vi "gyro-V5.vi"() -> ()   [LabVIEW 2017]
uses:
  lorentzian.ctl
  circle corners.ctl
  <vilib>/event_ctls.llb/eventvkey.ctl
  peak -- parameters -- complex fit.ctl
  wavepacket.ctl
  filter method control.ctl
  cursor winow.ctl
  parameters -- scan monitor control.ctl
  pid -- parameters.ctl
  agregator -- action.ctl
  filename-pattern.ctl
  plot refs -- filter related.ctl
  cursor window action.ctl
  cursor action.ctl
  KM_file -- read-write control.ctl
  filename-action.ctl
  publisher action.ctl
  MFLI controller action.ctl
  sweep parameters.ctl
  file -- read-write control.ctl
  <vilib>/Analysis/baseanly.llb/A x B.vi
  <vilib>/Analysis/baseanly.llb/Complex A x B.vi
  line -- complex.vi
  Q -- check range -- i -- integer.vi
  linear interpolation - real.vi
  linear interpolation iiii- complex.vi
  Q - not nan -- real.vi
  filter - complex - four.vi
  peak -- PM find lorenzian - V3.vi
  Q - not nan -- integer.vi
  tale of three indices.vi
  filter -- window span logic.vi
  linear interp iiii- complex - z-omega - divide.vi
  containing bix.vi
  peak -- guess at omega -- dzdomega V2.vi
  command stack.vi
  tale of three indices -- check state.vi
  peak -- z center from mult phase points.vi
  peak -- estimate for lorentzian.vi
  peak -- fake phase around center.vi
  peak -- get weights.vi
  peak -- four corner circle transformation logic.vi
  peak - fit phase around center - V2.vi
  array - generate range.vi
  circle center from three points.vi
  <vilib>/Utility/error.llb/Clear Errors.vi
  <vilib>/Analysis/Matrix/Numeric/Conversions/Array To Matrix.vi
  <vilib>/Analysis/Matrix/Numeric/Conversions/Array To Matrix - RA2.vi
  <vilib>/Analysis/baseanly.llb/Inverse Matrix.vi
  <vilib>/Analysis/baseanly.llb/Real Inverse Matrix.vi
  peak -- fit function -- minus arctan.vi
  <vilib>/gmath/NumericalOptimization/Nonlinear Curve Fit.vi
  <vilib>/gmath/NumericalOptimization/Nonlinear Curve Fit LM.vi
  KM_filter pipe - plot staff - more - V3.vi
  four-corner circle transformation.ctl
panel:
  out "read freq (Hz)":dbl=43834.543279430705 format="%-#11_11f"
  in  "all":enum32{"all", "other"}(tab)
  in  "subtract bgnd !":bool=TRUE
  out "angle (deg)":dbl format="%#11_11f"
  out "Temperature (K)":dbl=49.92548 format="%#11_11f"
  out "Field (T)":dbl=12.0 format="%#11_11f"
  out "Plot: circle sweep window":cluster{"all rows":dbl[], "all rows":dbl[]}[](graph)
  out "Plot: frequency shift vs T":cluster{dbl[], dbl[]}(graph)
  in  "MFLI mode":T1(tab)
  out "fit is fine":bool=TRUE
  in  "gamma factor":dbl=1.6
  in  "Auto-update sweep window!":bool
  in  "scan type":enum16{"linear", "arctan"}(ring)
  in  "N":i64=257
  out "sweep time (sec)":dbl=0.07489956999779679
  in  "control sweep!":bool
  out "circle frequency (Hz)":dbl=1234494.459530083 format="%#11_11f"
  out "circle gamma (Hz)":dbl=51497.57560712996 format="%#11_11f"
  out "circle phase (rad)":dbl=2.6250942279275566 format="%#11_11f"
  out "circle Q":dbl=23.971894695546876 format="%#11_11f"
  in  "history length":i32=5
  in  "delay-circle(msec)":i64
  out "read Voltage (V)":cdb=8.437092120710226e-06+0.006122499694529841i format="%#10_10f"
  in  "read !":bool
  out "read Voltage X (V)":dbl=8.437092120710226e-06 format="%#11_11f"
  out "read Voltage Y (V)":dbl=0.006122499694529841 format="%#11_11f"
  in  "delay-read (msec)":i64=300
  in  "read file":path=path "/Users/arkady/Desktop/local_data/Dec2017--preparing-for-Hybrid/sp030_122217.ASC"
  in  "read from disk":bool
  in  "reqested size":i64=30
  in  "refresh":bool=TRUE
  in  "PID parameters":T2={"P (sec)"=60.0, "I (sec)"=10.0}
  in  "save data":enum32{"save", "save num to dropbox"}(tab)
  out "data name pattern":T3={"prefix"="_empty_lever_", "group"="d"}
  out "freqsweep pattern":T3={"prefix"="lsco2", "group"="f"}
  in  "save data ?":bool
  in  "data file name":string="d001_empty_lever_122317.dat"
  in  "Save folder":path=path "/Users/arkady/Downloads"
  in  "freq sweep file name":string="f027_lsco2_122317.dat"
  in  "save number to dropbox":enum32{"save", "do not save"}(tab)
  in  "read file name":string="r003_silicon_empty_lever_122017.dat"
  in  "Save read folder":path=path "/Users/arkady/Downloads"
  out "left freq (Hz)":dbl=1189281.7830129303
  out "right freq (Hz)":dbl=1228830.8938969919
  in  "horisontal axis":enum16{"Time", "temperature", "field", "angle"}(ring)=enum."temperature"
  in  "vertical axis":T4(ring)
  out "center freq (Hz)":dbl=1209056.338454961
  out "window  (Hz)":dbl=39549.11088406133
  in  "talk to MFLI !":bool=TRUE
  in  "plot frequency shift":enum32{"plot"}(tab)
  in  "Plot frequency shift":bool
  in  "aggregate every # sec":dbl=1.0
  in  "plot length (min)":dbl=100.0
  out "Plot: frequency shift vs T 4":cluster{dbl[], dbl[]}(graph)
  out "Plot: frequency shift vs T 5":cluster{i32[], "Array":dbl[]}(graph)
  out "Plot: frequency shift vs T 2":cluster{dbl[], dbl[]}(graph)={[-1.2847105611270713e-06, -8.96090687489996e-07, -1.1878113186140714e-06, -1.0577364834927965e-06, -1.5485833177118755e-06, -1.2397929198806674e-06, -1.3595641386431873e-06, -1.95544238796184e-06, -1.8034552812236216e-06, -2.179156763955588e-06, -3.122427320687229e-06, -2.8927681404839808e-06, -3.2606669096266067e-06, -3.4335859766558394e-06, -4.275106687632253e-06, -4.265556221219542e-06, -4.306275487364196e-06, -5.474328117771029e-06, -5.250873166830706e-06, -6.158584714145268e-06, -6.308121182987117e-06, -6.715358985348123e-06, -7.0693959466281e-06, -7.254226550276167e-06, -7.471558204043555e-06, -8.180360377818478e-06, -8.644635949920024e-06, -9.450401470204308e-06, -1.0542161519072343e-05, -1.0662496796273006e-05, -1.1774006071250966e-05, -1.2809682001462881e-05, -1.3388752026600543e-05, -1.3901539528835397e-05, -1.577875366340369e-05, -1.6275815692673765e-05, -1.7367311318108792e-05, -1.8322241284696204e-05, -1.939577161026033e-05, -2.115027501101159e-05, -2.206547957836183e-05, -2.280844162782534e-05, -2.4123185115153962e-05, -2.3719380386582883e-05, -2.1949158634554497e-05, -1.7482795415692865e-05, -1.190476009852551e-05, -3.0012581586913445e-06, 6.6591691413936944e-06, 1.4913986718231652e-05, 2.1608211101800334e-05, 2.4441429222012755e-05, 2.5496538170609067e-05, 2.5006558977858244e-05, 2.47084954682896e-05, 2.3205579756867926e-05, 2.2241491423599197e-05, 2.059353741490501e-05, 1.940930308820722e-05, 1.8035523877789703e-05, 1.6795019444131693e-05, 1.6233689318685545e-05, 1.530601912625958e-05, 1.471481346136583e-05, 1.3668746476334144e-05, 1.278914735524648e-05, 1.1961636965375277e-05, 1.148511101983816e-05, 1.038015177533868e-05, 1.055813470630652e-05, 8.946114686992878e-06, 9.252763324432675e-06, 9.261580911233215e-06, 8.32864546005932e-06, 7.550850612980853e-06, 7.659009848135973e-06, 6.564878336519785e-06, 6.828313841636074e-06, 6.028961228097367e-06, 6.074863784114649e-06, 5.087873216594783e-06, 5.533364081213274e-06, 5.085350335296872e-06, 4.637182878582281e-06, 4.339275810721466e-06, 3.7404983334720106e-06, 3.8016720277973716e-06, 2.9030355925414103e-06, 3.3221723271601737e-06, 2.724834743267001e-06, 3.0361409970562057e-06, 2.469938271454002e-06, 2.1916218680781524e-06, 1.473344438791089e-06, 1.5465747082434236e-06, 1.5291782659004455e-06, 1.3674315612440997e-06, 9.633298642757269e-07, 8.898825337811226e-07], [-5.351696133733621e-06, -3.690354306686691e-06, -3.6817845026587138e-06, -3.6304954766072717e-06, -3.2238464103788782e-06, -3.732378935963822e-06, -3.493875482979771e-06, -3.3228636578776652e-06, -3.5305288089255853e-06, -3.7648610315931326e-06, -3.97228399037134e-06, -3.69199555481082e-06, -3.702050829314118e-06, -3.6362897452965515e-06, -4.059309516809881e-06, -3.708125867376757e-06, -3.8934710007503085e-06, -3.920425505771773e-06, -3.8396731962881915e-06, -4.145539651931423e-06, -4.426868555366925e-06, -5.042368648209767e-06, -4.738746005563639e-06, -4.890549160081816e-06, -5.391544637503511e-06, -5.223768648790353e-06, -5.325388776256424e-06, -5.912529897926599e-06, -6.493781160800396e-06, -6.198776272723992e-06, -7.250361850269486e-06, -7.26192304305288e-06, -7.774332746184141e-06, -8.356818571969059e-06, -9.494659847987037e-06, -9.933186332652295e-06, -1.0866378585117719e-05, -1.2559721845876861e-05, -1.4157112461896858e-05, -1.656537642835046e-05, -1.936170396817286e-05, -2.2793543082063973e-05, -2.6692434310764325e-05, -3.194302075894453e-05, -3.767957435737811e-05, -4.424063928058543e-05, -4.980677556288027e-05, -5.2904900834404434e-05, -5.2259193151987076e-05, -4.837844245967899e-05, -4.2136497452806694e-05, -3.570466251887759e-05, -3.0332314166196737e-05, -2.6071508393447144e-05, -2.1180215381563472e-05, -1.8286542839044908e-05, -1.61637622680976e-05, -1.3625750559341328e-05, -1.2108594610162641e-05, -1.0689795144437375e-05, -9.62045281676502e-06, -8.570007528029048e-06, -8.105558082533694e-06, -7.428892434368157e-06, -7.218695867625404e-06, -6.953805415589833e-06, -5.913334865014344e-06, -6.088309429175753e-06, -5.145987374849902e-06, -5.488187006895521e-06, -5.163517414643828e-06, -5.079842929772351e-06, -5.245282954840261e-06, -4.660283528196666e-06, -4.4589258860321075e-06, -4.13807438954911e-06, -4.565262237593832e-06, -4.053552425555827e-06, -3.4974249873645082e-06, -3.913051273651945e-06, -3.89264048603008e-06, -3.6773922014571442e-06, -3.2426624479706957e-06, -3.419821634783878e-06, -3.3651012599037013e-06, -3.573387544637086e-06, -4.131232704147514e-06, -3.2305802189117116e-06, -3.021417984572191e-06, -3.2398605602097806e-06, -3.508439835095558e-06, -3.546989372643574e-06, -3.729083758383661e-06, -3.2473817592994867e-06, -3.29870731020323e-06, -3.3620259083252726e-06, -3.419602935105049e-06, -4.225308611898116e-06, -3.737346070152369e-06]}
  out "Plot: frequency shift vs T 3":cluster{i32[], dbl[]}(graph)={[0, 1, 2, 3, 4, 5, 6, 7, 8, 9, 10, 11, 12, 13, 14, 15, 16, 17, 18, 19, 20, 21, 22, 23, 24, 25, 26, 27, 28, 29, 30, 31, 32, 33, 34, 35, 36, 37, 38, 39, 40, 41, 42, 43, 44, 45, 46, 47, 48, 49, 50, 51, 52, 53, 54, 55, 56, 57, 58, 59, 60, 61, 62, 63, 64, 65, 66, 67, 68, 69, 70, 71, 72, 73, 74, 75, 76, 77, 78, 79, 80, 81, 82, 83, 84, 85, 86, 87, 88, 89, 90, 91, 92, 93, 94, 95, 96, 97, 98], [-0.23559860043831193, -0.23820939062512414, -0.3120762913359678, -0.2835001183703665, -0.44780658796424877, -0.32070526654251785, -0.37109881260414546, -0.5319066481282504, -0.4722639722623221, -0.524696373474268, -0.6661788735811576, -0.6646137200418041, -0.7220903993361305, -0.7567345405074919, -0.8112846755002696, -0.8551933851256885, -0.8356992634466227, -0.9493152294582043, -0.9394070576242828, -0.9783311582294316, -0.9588814811243913, -0.9267379794474269, -0.9802698763137818, -0.9776201855738149, -0.9457143265769079, -1.0024951473096775, -1.0186705422504727, -1.0117383851591542, -1.0187082032726575, -1.0441935724590885, -1.0188444902666154, -1.0550639642963695, -1.0447176937736993, -1.0295365240674577, -1.0291006014399389, -1.0228351916589804, -1.0117082035896368, -0.9698748205564658, -0.9402791409053437, -0.9063694667492768, -0.8505714661765986, -0.7857248716608289, -0.7348809545553663, -0.6387178563870073, -0.5274684440579174, -0.37634000181515215, -0.2346170964234171, -0.05666856473380277, 0.12674275046362427, 0.29903345155814187, 0.4738466551438263, 0.6002776366427447, 0.6989959497442624, 0.7645517375308588, 0.8621349432337582, 0.9034008935958421, 0.9423491262817814, 0.9862736125756424, 1.0130206638602015, 1.035756014091886, 1.050605066301123, 1.0850669404773998, 1.083776083480046, 1.1032698129216518, 1.0849090392836143, 1.0727819505921015, 1.1116722316992618, 1.0833561407376393, 1.1105523962821076, 1.0914293641785555, 1.0473253514157124, 1.0687148941515687, 1.0554881441119783, 1.060651558581904, 1.0373768137660564, 1.0754397797680961, 0.9631595802552361, 1.0350672662925295, 1.0451346582720782, 0.9985529870514799, 0.9177123734459048, 0.984236082337904, 1.0031536192825101, 0.9353574049208152, 0.9111749823496003, 0.8082426158031351, 0.7438785320162125, 0.7320472832267922, 0.8327734332640132, 0.6992660900455262, 0.7133566540037093, 0.6082706202737593, 0.5313341296869087, 0.42592845813496805, 0.438412524592966, 0.42687019592046394, 0.38040311101033075, 0.22415893312212232, 0.2337528615998219]}
  in  "aggregator action":T5
  in  "Tab : everything":T6(tab)
  in  "Tab :  Fit controls":enum32{"complex plane", "complex plane 2"}(tab)
  in  "some":dbl=3172.0
  in  "Plot: fragment - filter":cluster{dbl[], dbl[]}[](graph)=[{array[18251 elements], array[18251 elements]}, {array[18251 elements], array[18251 elements]}, {array[18251 elements], array[18251 elements]}, {array[18251 elements], array[18251 elements]}]
  in  "scale gauge: Plot: complex plane - filter":dbl(slide)=0.00015000000000000001 min=0.0 max=0.3 step=1e-05 scale=0.0001..0.3 scale format="%#_5g"
  in  "Plot: complex plane - filter":cluster{dbl[], dbl[]}[](graph)=[{array[18251 elements], array[18251 elements]}, {array[18251 elements], array[18251 elements]}, {[1.0902546658046695e-05, 1.0889761640892542e-05, 1.0851457046051869e-05, 1.078778404426081e-05, 1.0698993923768004e-05, 1.058543709861469e-05, 1.044756172571057e-05, 1.0285911936163232e-05, 1.0101125687841252e-05, 9.89393224764595e-06, 9.6651493134281e-06, 9.41567978690808e-06, 9.146508210335277e-06, 8.858696880949628e-06, 8.55338165857973e-06, 8.231767482923022e-06, 7.895123618199276e-06, 7.5447786439446085e-06, 7.182115211715007e-06, 6.808564588392319e-06, 6.425601007627753e-06, 6.03473585171517e-06, 5.637511686855652e-06, 5.235496175353443e-06, 4.830275888769022e-06, 4.423450046446e-06, 4.016624204122979e-06, 3.6114039175385575e-06, 3.209388406036347e-06, 2.81216424117683e-06, 2.4212990852642467e-06, 2.038335504499682e-06, 1.6647848811769937e-06, 1.3021214489473908e-06, 9.517764746927217e-07, 6.151326099689789e-07, 2.935184343122684e-07, -1.1796788057628133e-08, -2.996081174432771e-07, -5.687796940160799e-07, -8.182492205360993e-07, -1.047032154753949e-06, -1.2542255949492504e-06, -1.439011843271231e-06, -1.6006616328185704e-06, -1.73853700572269e-06, -1.8520938308760026e-06, -1.9408839513688086e-06, -2.0045569531598684e-06, -2.0428615480005406e-06, -2.055646565154694e-06, -2.0428615480005406e-06, -2.0045569531598684e-06, -1.9408839513688077e-06, -1.8520938308760026e-06, -1.7385370057226892e-06, -1.6006616328185688e-06, -1.43901184327123e-06, -1.2542255949492496e-06, -1.0470321547539481e-06, -8.182492205360985e-07, -5.687796940160773e-07, -2.9960811744327624e-07, -1.1796788057627286e-08, 2.935184343122701e-07, 6.151326099689776e-07, 9.517764746927255e-07, 1.3021214489473916e-06, 1.664784881176997e-06, 2.038335504499683e-06, 2.4212990852642467e-06, 2.812164241176833e-06, 3.2093884060363485e-06, 3.6114039175385617e-06, 4.01662420412298e-06, 4.423450046446e-06, 4.8302758887690245e-06, 5.235496175353443e-06, 5.637511686855656e-06, 6.034735851715172e-06, 6.425601007627752e-06, 6.8085645883923205e-06, 7.182115211715006e-06, 7.544778643944612e-06, 7.895123618199278e-06, 8.231767482923025e-06, 8.553381658579734e-06, 8.858696880949628e-06, 9.146508210335279e-06, 9.41567978690808e-06, 9.665149313428104e-06, 9.893932247645952e-06, 1.0101125687841252e-05, 1.0285911936163232e-05, 1.0447561725710571e-05, 1.0585437098614693e-05, 1.0698993923768004e-05, 1.078778404426081e-05, 1.0851457046051869e-05, 1.0889761640892542e-05], [3.0357756803340517e-06, 3.442601522657073e-06, 3.847821809241494e-06, 4.249837320743704e-06, 4.647061485603221e-06, 5.037926641515804e-06, 5.42089022228037e-06, 5.7944408456030584e-06, 6.1571042778326605e-06, 6.507449252087329e-06, 6.844093116811073e-06, 7.165707292467784e-06, 7.47102251483768e-06, 7.758833844223328e-06, 8.028005420796131e-06, 8.277474947316151e-06, 8.506257881534001e-06, 8.713451321729303e-06, 8.898237570051283e-06, 9.059887359598623e-06, 9.19776273250274e-06, 9.311319557656056e-06, 9.400109678148862e-06, 9.46378267993992e-06, 9.502087274780593e-06, 9.514872291934746e-06, 9.502087274780593e-06, 9.46378267993992e-06, 9.40010967814886e-06, 9.311319557656056e-06, 9.19776273250274e-06, 9.059887359598621e-06, 8.898237570051283e-06, 8.713451321729302e-06, 8.506257881534001e-06, 8.277474947316151e-06, 8.028005420796131e-06, 7.758833844223327e-06, 7.4710225148376794e-06, 7.165707292467782e-06, 6.844093116811075e-06, 6.507449252087329e-06, 6.15710427783266e-06, 5.794440845603057e-06, 5.420890222280368e-06, 5.0379266415158025e-06, 4.647061485603221e-06, 4.249837320743704e-06, 3.847821809241493e-06, 3.4426015226570715e-06, 3.0357756803340496e-06, 2.62894983801103e-06, 2.2237295514266096e-06, 1.8217140399243985e-06, 1.4244898750648805e-06, 1.033624719152297e-06, 6.506611383877313e-07, 2.7711051506504534e-07, -8.55529171645576e-08, -4.3589789141922626e-07, -7.72541756142972e-07, -1.0941559317996812e-06, -1.399471154169577e-06, -1.687282483555225e-06, -1.9564540601280286e-06, -2.205923586648048e-06, -2.4347065208658994e-06, -2.6418999610611992e-06, -2.8266862093831814e-06, -2.9883359989305192e-06, -3.126211371834638e-06, -3.2397681969879523e-06, -3.3285583174807574e-06, -3.3922313192718172e-06, -3.4305359141124894e-06, -3.443320931266643e-06, -3.4305359141124894e-06, -3.3922313192718172e-06, -3.3285583174807565e-06, -3.2397681969879514e-06, -3.126211371834639e-06, -2.9883359989305175e-06, -2.8266862093831797e-06, -2.6418999610611975e-06, -2.434706520865897e-06, -2.2059235866480456e-06, -1.956454060128026e-06, -1.687282483555225e-06, -1.3994711541695744e-06, -1.0941559317996795e-06, -7.72541756142967e-07, -4.358978914192233e-07, -8.555291716455718e-08, 2.771105150650479e-07, 6.506611383877338e-07, 1.033624719152303e-06, 1.4244898750648839e-06, 1.821714039924399e-06, 2.2237295514266125e-06, 2.628949838011031e-06]}, {[-1.0628665430958349e-06, 6.164050781399584e-07, 1.2136346376816573e-06], [-2.749099041575702e-07, -4.987758850147442e-07, 3.798056853807086e-07]}, {[-2.689773598781885e-07, -2.658273840778637e-07, -2.626774082775389e-07, -2.595274324772141e-07, -2.5637745667688934e-07, -2.5322748087656455e-07, -2.5007750507623977e-07, -2.46927529275915e-07, -2.437775534755902e-07, -2.406275776752654e-07, -2.3747760187494066e-07, -2.3432762607461587e-07, -2.311776502742911e-07, -2.280276744739663e-07, -2.2487769867364152e-07, -2.2172772287331676e-07, -2.1857774707299197e-07, -2.154277712726672e-07, -2.122777954723424e-07, -2.0912781967201762e-07], [-2.2381592717709463e-07, -2.1935795690029337e-07, -2.1489998662349214e-07, -2.1044201634669088e-07, -2.0598404606988962e-07, -2.015260757930884e-07, -1.9706810551628713e-07, -1.926101352394859e-07, -1.8815216496268464e-07, -1.8369419468588339e-07, -1.7923622440908216e-07, -1.747782541322809e-07, -1.7032028385547964e-07, -1.658623135786784e-07, -1.6140434330187715e-07, -1.569463730250759e-07, -1.5248840274827466e-07, -1.480304324714734e-07, -1.4357246219467214e-07, -1.3911449191787091e-07]}, {[6.164050781399584e-07, 7.064288860098442e-07, 7.9645269387973e-07, 8.86476501749616e-07, 9.765003096195017e-07, 1.0665241174893877e-06, 1.1565479253592736e-06, 1.2465717332291596e-06, 1.3365955410990453e-06, 1.426619348968931e-06, 1.516643156838817e-06, 1.606666964708703e-06, 1.696690772578589e-06, 1.7867145804484747e-06, 1.8767383883183606e-06, 1.9667621961882463e-06, 2.0567860040581323e-06, 2.1468098119280182e-06, 2.2368336197979038e-06, 2.32685742766779e-06], [-4.987758850147442e-07, -4.987758850147442e-07, -4.987758850147442e-07, -4.987758850147442e-07, -4.987758850147442e-07, -4.987758850147442e-07, -4.987758850147442e-07, -4.987758850147442e-07, -4.987758850147442e-07, -4.987758850147442e-07, -4.987758850147442e-07, -4.987758850147442e-07, -4.987758850147442e-07, -4.987758850147442e-07, -4.987758850147442e-07, -4.987758850147442e-07, -4.987758850147442e-07, -4.987758850147442e-07, -4.987758850147442e-07, -4.987758850147442e-07]}]
  out "Plot: dz/domega":cluster{"omega out":dbl[], dbl[]}(graph)
  out "Plot: win omega":T7(graph)
  out "Plot: phase":cluster{"omega out":dbl[], dbl[]}(graph)
  out "Plot: phase around center":cluster{dbl[], dbl[]}[](graph)
  out "Plot: fragment":cluster{dbl[], dbl[]}[](graph)
  out "Plot: complex plane":cluster{dbl[], dbl[]}[](graph)=[{array[18251 elements], array[18251 elements]}, {[4.093261515777318e-06, 4.09109240444531e-06, 4.084619278630759e-06, 4.073944223394617e-06, 4.059235590734925e-06, 4.040725344575241e-06, 4.018705402554987e-06, 3.993523032313897e-06, 3.965575374873894e-06, 3.9353031814879255e-06, 3.903183862729422e-06, 3.869723959442356e-06, 3.835451154289541e-06, 3.8009059498818182e-06, 3.7666331447290027e-06, 3.7331732414419364e-06, 3.701053922683433e-06, 3.670781729297465e-06, 3.6428340718574613e-06, 3.6176517016163716e-06, 3.5956317595961173e-06, 3.5771215134364333e-06, 3.5624128807767425e-06, 3.5517378255406e-06, 3.5452646997260484e-06, 3.543095588394041e-06, 3.5452646997260484e-06, 3.5517378255406e-06, 3.5624128807767425e-06, 3.5771215134364333e-06, 3.5956317595961173e-06, 3.6176517016163716e-06, 3.6428340718574613e-06, 3.670781729297465e-06, 3.701053922683433e-06, 3.7331732414419364e-06, 3.766633144729003e-06, 3.8009059498818182e-06, 3.835451154289541e-06, 3.869723959442356e-06, 3.903183862729422e-06, 3.9353031814879255e-06, 3.965575374873894e-06, 3.993523032313897e-06, 4.018705402554987e-06, 4.040725344575242e-06, 4.059235590734925e-06, 4.073944223394617e-06, 4.084619278630759e-06, 4.09109240444531e-06], [3.4730573631850562e-06, 3.507534400522981e-06, 3.5414677143865035e-06, 3.574322156145216e-06, 3.605579591626292e-06, 3.634747072399907e-06, 3.661364609870454e-06, 3.6850124295714753e-06, 3.7053175912597633e-06, 3.7219598704057783e-06, 3.734676808325772e-06, 3.7432678513120154e-06, 3.747597513484575e-06, 3.747597513484575e-06, 3.7432678513120154e-06, 3.734676808325772e-06, 3.7219598704057783e-06, 3.7053175912597633e-06, 3.6850124295714753e-06, 3.661364609870454e-06, 3.634747072399907e-06, 3.6055795916262915e-06, 3.574322156145216e-06, 3.5414677143865035e-06, 3.507534400522981e-06, 3.4730573631850562e-06, 3.4385803258471313e-06, 3.404647011983609e-06, 3.371792570224896e-06, 3.3405351347438205e-06, 3.311367653970205e-06, 3.2847501164996586e-06, 3.261102296798637e-06, 3.240797135110349e-06, 3.224154855964334e-06, 3.2114379180443405e-06, 3.202846875058097e-06, 3.1985172128855375e-06, 3.1985172128855375e-06, 3.202846875058097e-06, 3.2114379180443405e-06, 3.224154855964334e-06, 3.240797135110349e-06, 3.2611022967986376e-06, 3.284750116499659e-06, 3.3113676539702056e-06, 3.3405351347438205e-06, 3.3717925702248966e-06, 3.404647011983609e-06, 3.4385803258471313e-06]}, {[3.6823320311784962e-06, 3.6959166832692147e-06, 3.7095013353599328e-06, 3.7230859874506512e-06, 3.7366706395413693e-06, 3.7502552916320878e-06, 3.7638399437228063e-06, 3.7774245958135243e-06, 3.791009247904243e-06, 3.804593899994961e-06, 3.818178552085679e-06, 3.831763204176397e-06, 3.845347856267116e-06, 3.858932508357834e-06, 3.872517160448552e-06, 3.886101812539271e-06, 3.899686464629989e-06, 3.9132711167207074e-06, 3.9268557688114255e-06, 3.940440420902144e-06], [3.233857949158204e-06, 3.257777890560889e-06, 3.2816978319635747e-06, 3.3056177733662597e-06, 3.329537714768945e-06, 3.35345765617163e-06, 3.3773775975743154e-06, 3.4012975389770005e-06, 3.4252174803796856e-06, 3.449137421782371e-06, 3.4730573631850562e-06, 3.4969773045877413e-06, 3.520897245990427e-06, 3.544817187393112e-06, 3.568737128795797e-06, 3.5926570701984825e-06, 3.6165770116011676e-06, 3.6404969530038527e-06, 3.664416894406538e-06, 3.6883368358092233e-06]}, {[3.5789791380588267e-06, 3.602899079461512e-06, 3.6268190208641973e-06, 3.6507389622668824e-06, 3.674658903669568e-06, 3.698578845072253e-06, 3.722498786474938e-06, 3.7464187278776236e-06, 3.7703386692803087e-06, 3.7942586106829942e-06, 3.818178552085679e-06, 3.842098493488365e-06, 3.8660184348910495e-06, 3.889938376293735e-06, 3.9138583176964205e-06, 3.937778259099106e-06, 3.961698200501791e-06, 3.985618141904476e-06, 4.009538083307162e-06, 4.0334580247098464e-06], [3.608903884092239e-06, 3.595319232001521e-06, 3.5817345799108024e-06, 3.568149927820084e-06, 3.554565275729366e-06, 3.5409806236386478e-06, 3.5273959715479293e-06, 3.513811319457211e-06, 3.5002266673664928e-06, 3.4866420152757747e-06, 3.4730573631850562e-06, 3.4594727110943377e-06, 3.4458880590036197e-06, 3.4323034069129016e-06, 3.418718754822183e-06, 3.4051341027314647e-06, 3.3915494506407466e-06, 3.3779647985500286e-06, 3.36438014645931e-06, 3.3507954943685916e-06]}, {[0.11020964852293831, 0.1081676673664668, 0.10605808731817996, 0.10388222679693825, 0.10164144564474008, 0.09933714427686499, 0.09697076280665969, 0.09454378014551397, 0.0920577130785894, 0.08951411531687781, 0.08691457652618259, 0.08426072133362926, 0.0815542083123265, 0.07879672894481177, 0.07599000656593, 0.07313579528580517, 0.0702358788935788, 0.06729206974259966, 0.06430620761776203, 0.06128015858569991], [0.0803136449141255, 0.08304340836327952, 0.08572127459436578, 0.0883455700281582, 0.09091465456543511, 0.09342692261198808, 0.09588080408206583, 0.09827476537962686, 0.10060731035678701, 0.10287698124886316, 0.10508235958542876, 0.10722206707681159, 0.10929476647548003, 0.1112991624117792, 0.11323400220349483, 0.1150980766387388, 0.1168902207316674, 0.1186093144505593, 0.12025428341779912, 0.1218240995813284]}, {[0.12233229108551504, 0.12006569200183163, 0.11772405814823327, 0.11530885296965496, 0.11282158589071498, 0.11026381137237364, 0.10763712794044575, 0.104943177186574, 0.10218364274228772, 0.09936024922678786, 0.09647476116911617, 0.09352898190538197, 0.09052475245173591, 0.08746395035379456, 0.0843484885132358, 0.08118031399229725, 0.07796140679692595, 0.07469377863933911, 0.07137947168076934, 0.06802055725518039], [0.08914775705400713, 0.09217779448256808, 0.09515022599907384, 0.09806319393058342, 0.1009148777669608, 0.10370349529863458, 0.10642730373042088, 0.10908460077071364, 0.11167372569536141, 0.11419306038556593, 0.11664103033915374, 0.11901610565458869, 0.12131680198711066, 0.12354168147640275, 0.12568935364520709, 0.1277584762683279, 0.12974775621147863, 0.13165595023944865, 0.13348186579308485, 0.13522436173460234]}, {array[18251 elements], array[18251 elements]}]
  in  "scale gauge: Plot: complex plane":dbl(slide)=0.00025 min=0.0 max=0.3 step=1e-05 scale=0.0001..1.0 scale format="%#_2g"
  out "window width (kHz)":dbl=76.27809365793496
  out "window center (kHz)":dbl=3399.029286744401
  out "# of points in window":dbl=953.475933538175
  in  "use fast fit?":bool
  out "pm lorentzian":T8={"Amplitude"=0.014166105720943529, "omega(0)"=1234494.459530083, "Gamma"=51497.57560712996, "phase"=2.6250942279275566, "Q"=23.971894695546876, "Norm  Ampl"=nan, "z (inf)"=3.6823320311784962e-06+3.233857949158204e-06i, "4corners"={"z (-pi/2)"=3.5789791380588267e-06+3.608903884092239e-06i, "z(inf)"=3.6823320311784962e-06+3.233857949158204e-06i, "z (pi/2)"=4.057377966112532e-06+3.3372108422778735e-06i, "z center"=3.818178552085679e-06+3.4730573631850562e-06i, "z(0)"=3.9540250729928624e-06+3.7122567772119084e-06i, "radius"=2.750829636916383e-07}} {"z (inf)" format="%#9_9f"; "Q" format="%#9_9f"; "phase" format="%#9_9f"; "Gamma" format="%#9_9f"; "omega(0)" format="%#9_9f"}
  in  "plot staff":enum16{"plot", "do not plot", "a"}(ring)
  in  "fit?":bool=TRUE
  out "Freq out":dbl[](array[numeric])
  out "Voltage out":cdb[](array[numeric])
  in  "cursor bracket: fit boundaries":T10={"left"=1016786.9846609245, "right "=1413121.3581259316, "center"=1214954.171393428, "window"=396334.373465007, "cursors"=[3, 4, 5], "relative"=0, "absolute"=0, "fixed vertical offset"=0.0, "vertical offset"=0.0, "skew"=0.0, "default window frac"=0.1, "kind"=enum."symmetric", "skew.left"=0.5, "skew.right"=0.5, "Plot ref"=refnum, "wing order"=enum."forw"}
  in  "scan monitor control":T11={"gamma acc. frac. - min "=0.3, "gamma acc frac.. - max"=3.0, "peak acc. fraction (af)"=5.0, "min peak acc. window (kHz)"=0.5, "use"=enum."fraction", "abs gamma min(kHz)"=0.005, "abs gamma max(kHz)"=5.0, "# points"=5, "gamma-factor (fa)"=3.0, "interpolate"=enum."line", "init"=TRUE, "Unique strike parameters"=TRUE, "max peak acc. window (kHz)"=10.0, "spacing factor"=1.5, "iterate #"=1, "overwrite ctl?"=FALSE, "write _m files?"=FALSE, "max slope (kHz/sweep)"=0.5, "funnel state"=enum."funnel open"}
  in  "Update system parameters":bool
  in  "parameters: complex fit":T12={"main VI path"=path "", "scale factor"=3.0, "# of grid points"=200, "parameters: wavepacket"={"R"=0.5, "wave number"=22.0, "delta k"=7.0, "radii vector"=[], "radial section"=[], "wave vector"=22.0, "wavepacket is"=TRUE}, "span"=0.27789, "interference ?"=enum."cp z center", "filter method"=enum."three"} {"span" min=0.0 max=0.5 step=1e-05 scale=0.0001..0.5 scale format="%#_5f"; "parameters: wavepacket"."delta k" format="%#_3f"; "parameters: wavepacket"."wave number" format="%#_3f"; "parameters: wavepacket"."R" format="%#_3f"}
  in  "cursor bracket: circle window":T10={"left"=1189281.7830129303, "right "=1228830.8938969919, "center"=1209056.338454961, "window"=39549.11088406133, "cursors"=[0, 1, 2], "relative"=1, "absolute"=1, "fixed vertical offset"=0.0, "vertical offset"=0.0, "skew"=0.0, "default window frac"=0.1, "kind"=enum."symmetric", "skew.left"=0.5, "skew.right"=0.5, "Plot ref"=refnum, "wing order"=enum."forw"}
  in  "Tab : parameters":enum32{"Page 1"}(tab)
  out "VKey":T15
  out "Char":i16=45
  # "three strikes"
  # "search window"
  # "linear extrapolation"
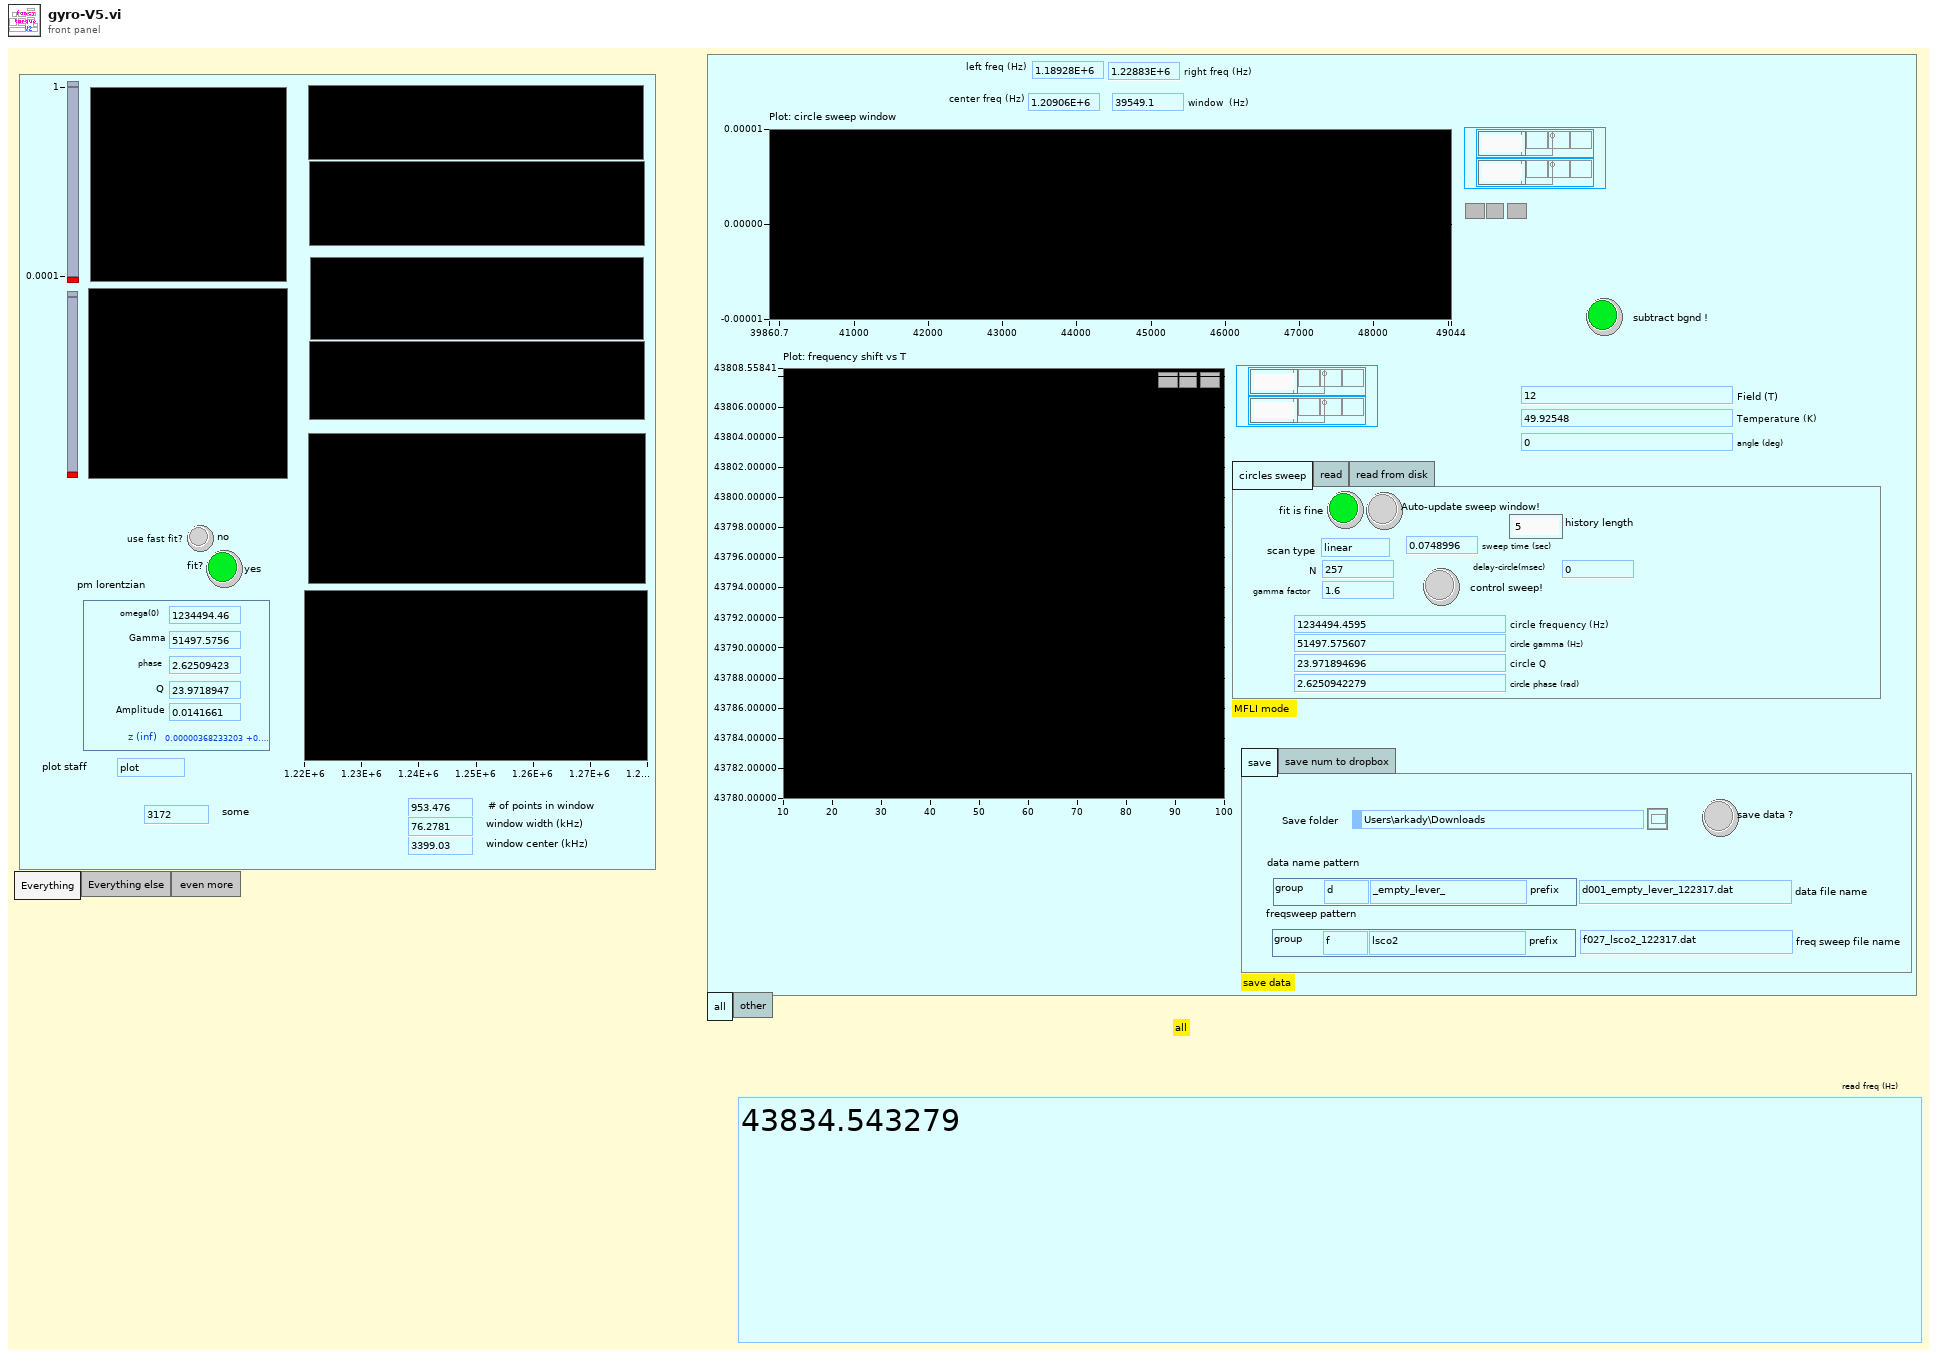
[diagram p1: front panel]
types:
  T1 = enum32{"circles sweep", "read", "read from disk", "circle PLL"}
  T2 = typedef "pid -- parameters.ctl" = cluster{"P (sec)":dbl, "I (sec)":dbl}
  T3 = typedef "filename-pattern.ctl" = cluster{"prefix":string, "group":string}
  T4 = enum16{"frequency", "gamma", "phase", "background"}
  T5 = typedef "agregator -- action.ctl" = enum16{"append", "interpolate", "empty!", "force", "init", "scale", "read last"}
  T6 = enum32{"Everything", "Everything else", "even more "}
  T7 = cluster{"omega out":dbl[], "win omega out":dbl[]}
  T8 = typedef "lorentzian.ctl" = cluster{"Amplitude":dbl, "omega(0)":dbl, "Gamma":dbl, "phase":dbl, "Q":dbl, "Norm  Ampl":dbl, "z (inf)":cdb, "4corners":T9}
  T9 = typedef "circle corners.ctl" = cluster{"z (-pi/2)":cdb, "z(inf)":cdb, "z (pi/2)":cdb, "z center":cdb, "z(0)":cdb, "radius":dbl}
  T10 = typedef "cursor winow.ctl" = cluster{"left":dbl, "right ":dbl, "center":dbl, "window":dbl, "cursors":i32[], "relative":i32, "absolute":i32, "fixed vertical offset":dbl, "vertical offset":dbl, "skew":dbl, "default window frac":dbl, "kind":enum16{"symmetric", "skewed", "fancy"}, "skew.left":dbl, "skew.right":dbl, "Plot ref":refnum<vi>, "wing order":enum16{"forw", "back"}}
  T11 = typedef "parameters -- scan monitor control.ctl" = cluster{"gamma acc. frac. - min ":dbl, "gamma acc frac.. - max":dbl, "peak acc. fraction (af)":dbl, "min peak acc. window (kHz)":dbl, "use":enum16{"window", "fraction"}, "abs gamma min(kHz)":dbl, "abs gamma max(kHz)":dbl, "# points":i32, "gamma-factor (fa)":dbl, "interpolate":enum16{"line", "last"}, "init":bool, "Unique strike parameters":bool, "max peak acc. window (kHz)":dbl, "spacing factor":dbl, "iterate #":i32, "overwrite ctl?":bool, "write _m files?":bool, "max slope (kHz/sweep)":dbl, "funnel state":enum16{"funnel open", "funnel closed"}}
  T12 = typedef "peak -- parameters -- complex fit.ctl" = cluster{"main VI path":path, "scale factor":dbl, "# of grid points":i32, "parameters: wavepacket":T13, "span":dbl, "interference ?":enum16{"cp z center", "pm zcenter", "fancy"}, "filter method":T14}
  T13 = typedef "wavepacket.ctl" = cluster{"R":dbl, "wave number":dbl, "delta k":dbl, "radii vector":dbl[], "radial section":cdb[], "wave vector":dbl, "wavepacket is":bool}
  T14 = typedef "filter method control.ctl" = enum16{"four", "five", "one", "two", "three", "zero", "minus one", "minus two"}
  T15 = typedef "eventvkey.ctl" = enum16{"ASCII", "Enter", "Return", "Shift", "Ctrl", "Alt", "Cmd", "Opt", "Caps", "NumLock", "Clear", "Break", "Up", "Down", "Left", "Right", "Insert", "Delete", "Home", "End", "PageUp", "PageDown", "Escape", "Help", "Pause", "ScrollLock", "F1", "F2", "F3", "F4", "F5", "F6", "F7", "F8", "F9", "F10", "F11", "F12", "F13", "F14", "F15", "F16", "F17", "F18", "F19", "F20", "F21", "F22", "F23", "F24", "Play", "VolumeUp", "VolumeDown", "Mute", "Two Byte Char"}
  T16 = typedef "cursor window action.ctl" = enum16{"balance", "h. offset change", "cursor moves", "change center", "change window", "init", "check", "reset", "set y to middle", "idle", "-write all Y", "-write left.X", "-write center.X", "-write right.X", "-write all X", "-change center", "-change window", "-change skew", "-read cursor 2", "-read cursor 1", "-read cursor 0", "-read all cursors", "-reset", "-read plot scale", "-set y to middle", "-Q: center.Y is visible", "-Q: window is visible", "-parse center.Y", "-right left from center", "-left move", "-right move", "-set center.Y", "-empty", "-set cursors to default", "-check", "-write center.Y", "-copy cursor 1", "-copy cursor 0", "-copy cursor 2", "move right", "move left", "shrink", "broaden", "skew up", "skew down", "-write plot scale", "zoom X", "change cen&win", "zoom to all data", "color--red", "color--green", "color--yellow", "read", "zoom out", "zoom in", "slide right", "slide left"}
  T17 = typedef "plot refs -- filter related.ctl" = cluster{"Plot: complex plane - filter":refnum<vi>, "Plot: dz/domega":refnum<vi>, "Plot: fragment filter":refnum<vi>, "Plot: win omega":refnum<vi>, "Plot: phase":refnum<vi>, "Plot: phase around center":refnum<vi>, "Plot: complex plane":refnum<vi>, "Plot: fragment":refnum<vi>}
  T18 = typedef "MFLI controller action.ctl" = enum16{"Initialize", "Scan frequency", "open", "close", "read", "circle PLL"}
  T19 = typedef "file -- read-write control.ctl" = enum16{"read", "write all", "append one line"}
  T20 = typedef "sweep parameters.ctl" = cluster{"scan type":enum16{"linear", "arctan"}, "N":i64, "cursor window":T10}
  T21 = typedef "cursor action.ctl" = enum16{"range", "read", "write", "check", "zoom out", "smart zoom out"}
  T22 = typedef "KM_file -- read-write control.ctl" = enum16{"read", "write all", "append one line"}
  T23 = typedef "filename-action.ctl" = enum16{"rewrite", "parse"}
  T24 = typedef "publisher action.ctl" = enum16{"set", "get"}
  T25 = typedef "four-corner circle transformation.ctl" = enum16{"z(c) z(inf)", "z(c) z(zero)", "fix phase", "calculate lorentzian", "z(0) z(+-pi/2)", "shift to zcenter", "to  canonical", "get canonical phase", "get4corners"}
  T26 = typedef "interpolation state - real.ctl" = cluster{"requested size":i32, "Array":dbl[], "actual number of elements":i32}
  T27 = typedef "interpolation state - complex.ctl" = cluster{"requested size":i32, "Array":cdb[], "actual number of elements":i32}
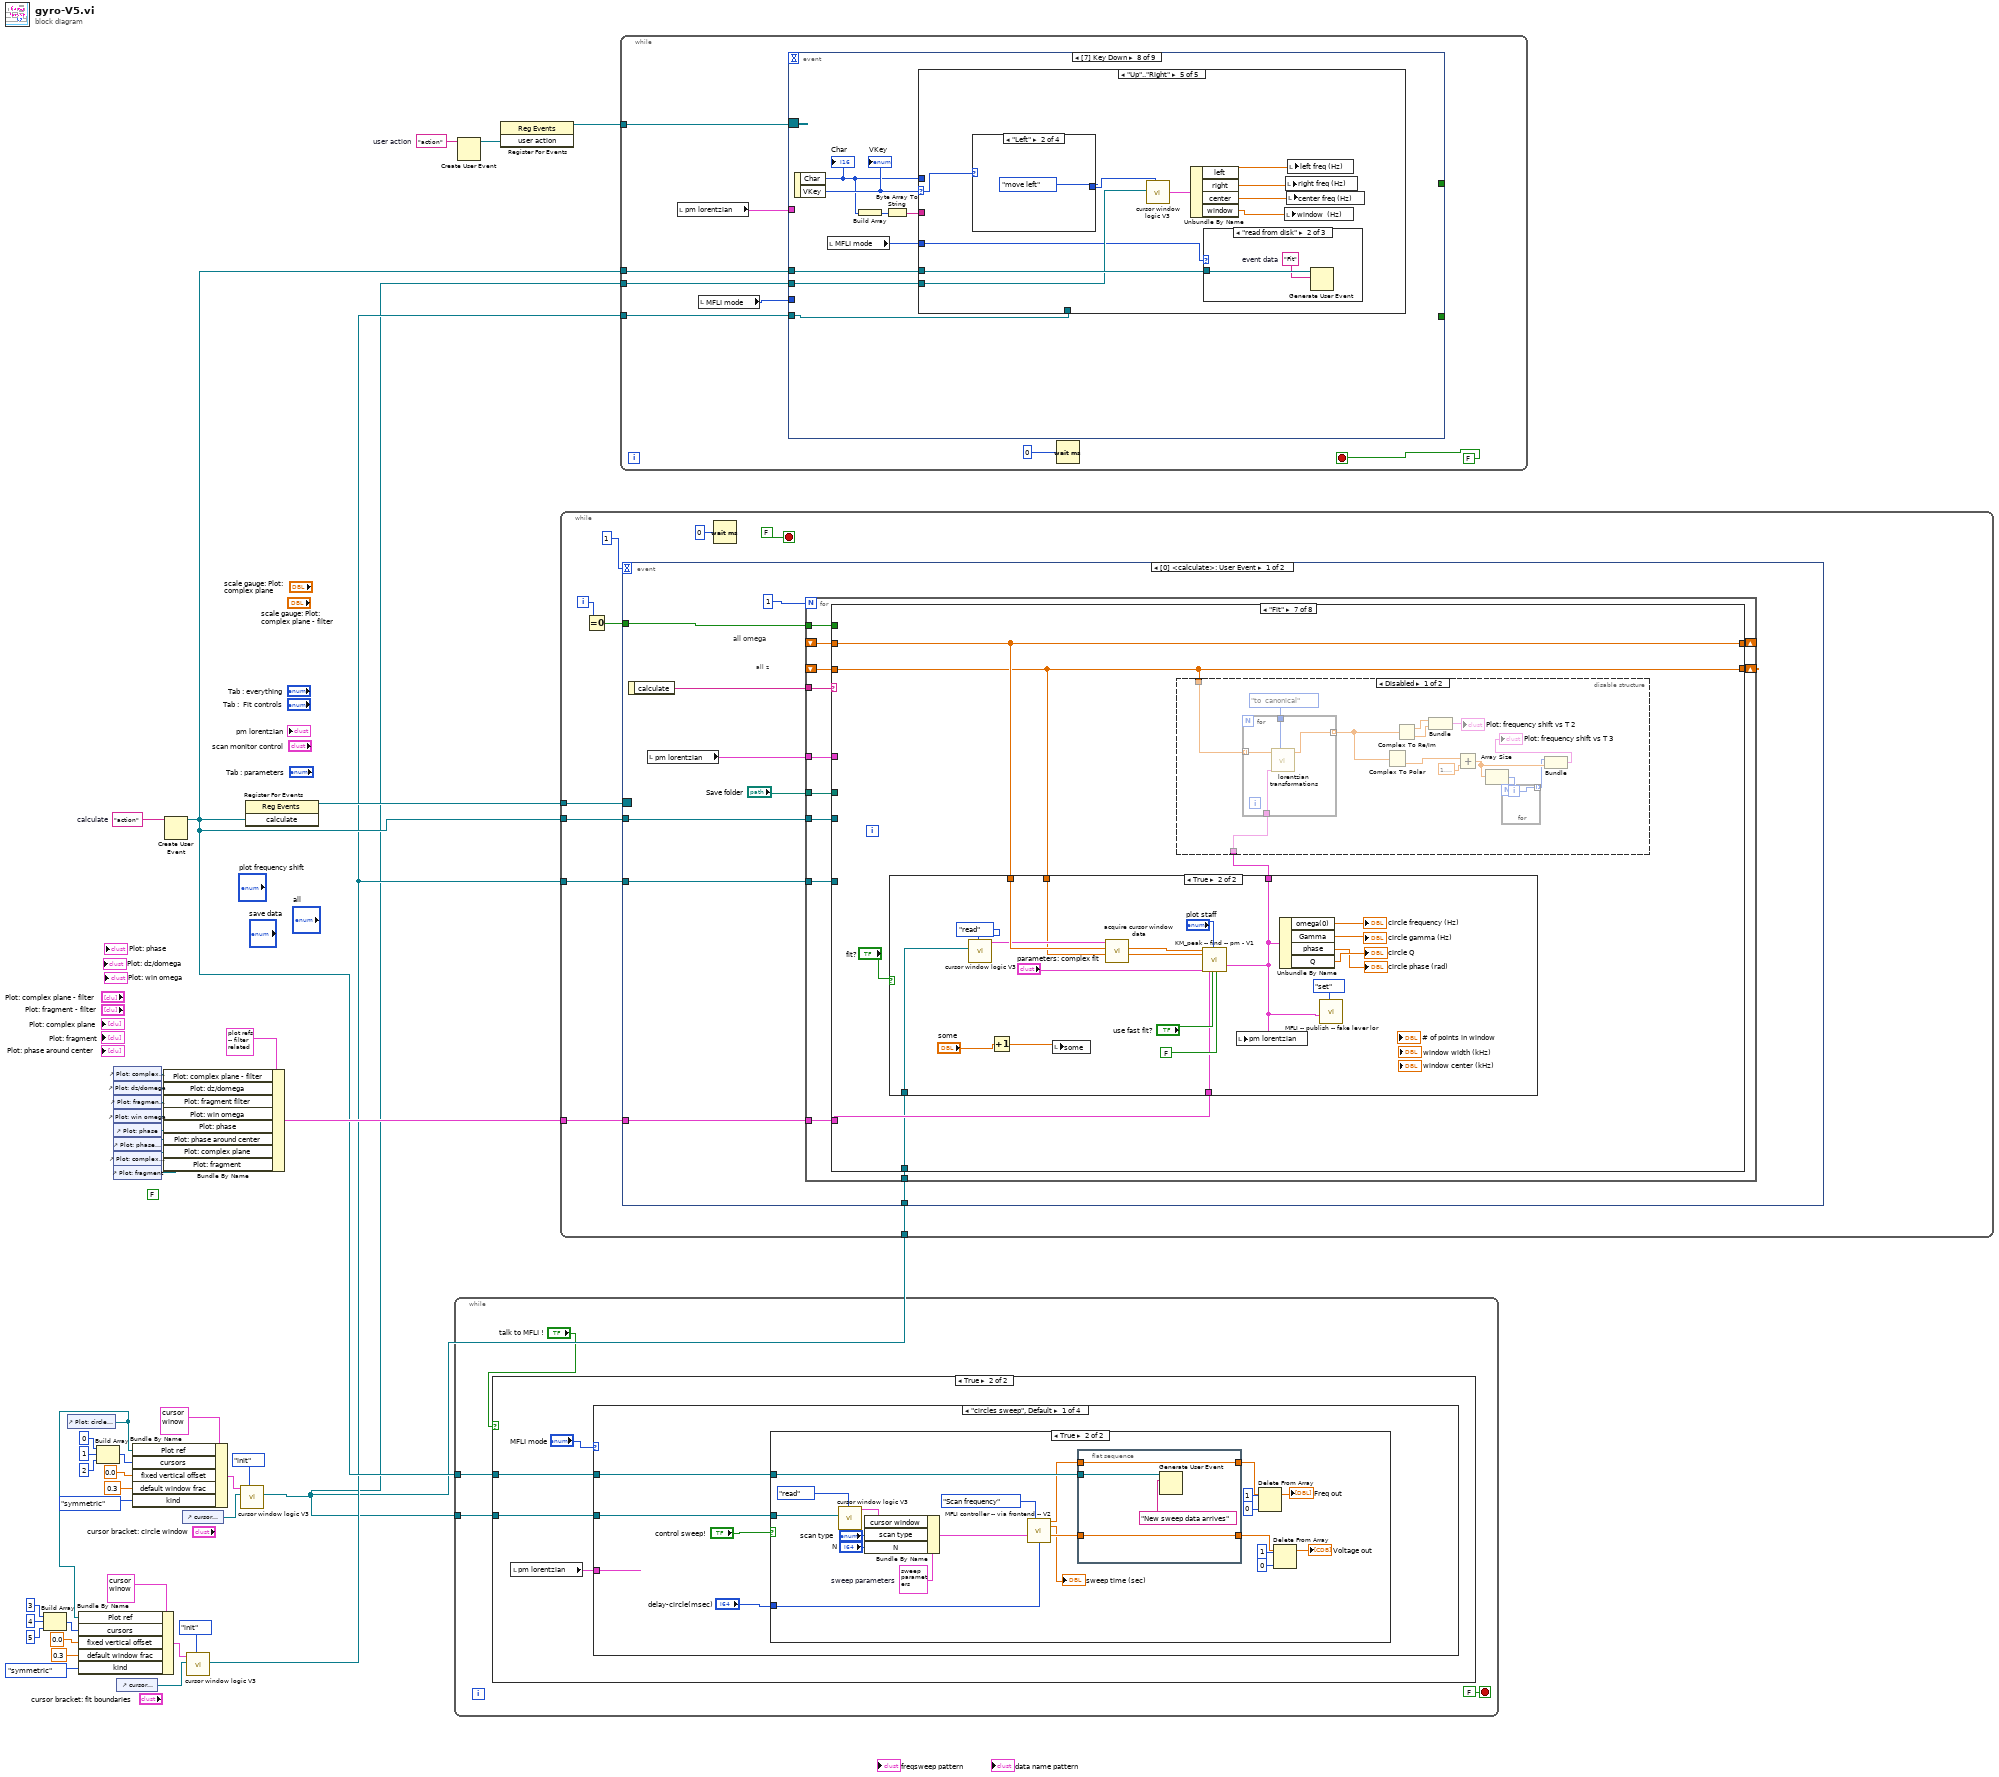
[diagram p0: block diagram]
diagram:
  w38 = "action"  # user action
  w40 = "action"  # calculate
  (unwired) FALSE
  n1 = Build Array(3, 4, 5) -> (w14:i32[])
  n2 = control-ref of="Plot: circle sweep window"() -> (w3:refnum<vi>)
  n3 = Bundle By Name(cluster=T10 {"left"=0.0, "right "=0.0, "center"=0.0, "window"=0.0, "cursors"=[], "relative"=0, "absolute"=0, "fixed vertical offset"=0.0, "vertical offset"=0.0, "skew"=0.0, "default window frac"=0.0, "kind"=enum."symmetric", "skew.left"=0.0, "skew.right"=0.0, "Plot ref"=refnum, "wing order"=enum."forw"} ("cursor bracket: All, data window"), "Plot ref"=w3, "cursors"=w14, "fixed vertical offset"=0.0, "default window frac"=0.3 ("fixed vertical offset"), "kind"=enum16{"symmetric", "skewed", "fancy"}."symmetric") -> (w6:T10)
  n4 = Build Array(0, 1, 2) -> (w25:i32[])
  n5 = control-ref of="Plot: complex plane - filter"() -> (w35:refnum<vi>)
  n6 = control-ref of="Plot: dz/domega"() -> (w34:refnum<vi>)
  n7 = control-ref of="Plot: fragment - filter"() -> (w33:refnum<vi>)
  n8 = control-ref of="Plot: win omega"() -> (w32:refnum<vi>)
  n9 = control-ref of="Plot: phase"() -> (w31:refnum<vi>)
  n10 = control-ref of="Plot: phase around center"() -> (w29:refnum<vi>)
  n11 = control-ref of="Plot: complex plane"() -> (w28:refnum<vi>)
  n12 = control-ref of="Plot: fragment"() -> (w27:refnum<vi>)
  n13 = control-ref of="cursor bracket: fit boundaries"() -> (w4:refnum<vi>)
  n14 = Bundle By Name(cluster=T10 {"left"=0.0, "right "=0.0, "center"=0.0, "window"=0.0, "cursors"=[], "relative"=0, "absolute"=0, "fixed vertical offset"=0.0, "vertical offset"=0.0, "skew"=0.0, "default window frac"=0.0, "kind"=enum."symmetric", "skew.left"=0.0, "skew.right"=0.0, "Plot ref"=refnum, "wing order"=enum."forw"} ("cursor bracket: All, data window"), "Plot ref"=w3, "cursors"=w25, "fixed vertical offset"=0.0, "default window frac"=0.3 ("fixed vertical offset"), "kind"=enum16{"symmetric", "skewed", "fancy"}."symmetric") -> (w17:T10)
  n15 = Bundle By Name(cluster=T17 {"Plot: complex plane - filter"=refnum, "Plot: dz/domega"=refnum, "Plot: fragment filter"=refnum, "Plot: win omega"=refnum, "Plot: phase"=refnum, "Plot: phase around center"=refnum, "Plot: complex plane"=refnum, "Plot: fragment"=refnum} ("plots: filter related"), "Plot: complex plane - filter"=w35, "Plot: dz/domega"=w34, "Plot: fragment filter"=w33, "Plot: win omega"=w32, "Plot: phase"=w31, "Plot: phase around center"=w29, "Plot: complex plane"=w28, "Plot: fragment"=w27) -> (w30:T17)
  n16 = Create User Event(user event datatype=w40) -> (user event=w26:refnum<user-event>)  [unwired: 1 in, 1 out]
  n17 = control-ref of="cursor bracket: circle window"() -> (w16:refnum<vi>)
  n18 = call "cursor window logic V3.vi"("cursor window action"=cursor_window_action."init", "cursor window in"=w4, "cursor window init"=w6) -> ("cursor window out"=w2:refnum<vi>)  [unwired: 7 in, 1 out]
  n19 = call "cursor window logic V3.vi"("cursor window action"=cursor_window_action."init", "cursor window in"=w16, "cursor window init"=w17) -> ("cursor window out"=w1:refnum<vi>)  [unwired: 7 in, 1 out]
  n20 = register-events(w26) -> (reference out=w41:refnum<event-registration>)  [unwired: 2 in, 1 out]
  n21 = while {
    tunnel: w26 -> [w45]
    tunnel: w1 -> [w43]
    stop <- FALSE stop-if-true
    n22 = case shown="True" "talk to MFLI !" {
      tunnel: w45 -> [_ w49]
      tunnel: w43 -> [_ w48]
      frame False {
      }
      frame True {
        n23 = local read "pm lorentzian"() -> (w46:T8)
        n24 = case shown="\"circles sweep\", Default" "MFLI mode" {
          tunnel: w49 -> [w53 w82 w109 w121]
          tunnel: w48 -> [w52 w81 _ _]
          tunnel: w46 -> [_ _ _ _]
          frame "circles sweep", Default {
            n25 = case shown="True" "control sweep!" {
              tunnel: w53 -> [_ w74]
              tunnel: w52 -> [_ w73]
              tunnel: "delay-circle(msec)" -> [_ w54]
              frame False {
              }
              frame True {
                w68 = T20 {"scan type"=enum."linear", "N"=-1, "cursor window"={"left"=2378.60310421286, "right "=2421.6740576496672, "center"=2421.6740576496672, "window"=2421.6740576496672, "cursors"=[], "relative"=0, "absolute"=0, "fixed vertical offset"=2421.6740576496672, "vertical offset"=2421.6740576496672, "skew"=2421.6740576496672, "default window frac"=2421.6740576496672, "kind"=enum."skewed", "skew.left"=2421.6740576496672, "skew.right"=2421.6740576496672, "Plot ref"=refnum, "wing order"=enum."back"}}  # sweep parameters
                n26 = call "cursor window logic V3.vi"("cursor window action"=cursor_window_action."read", "cursor window in"=w73) -> ("cursor window out"=w66:T10)  [unwired: 8 in, 1 out]
                n27 = Bundle By Name(cluster=w68, "cursor window"=w66, "scan type"="scan type", "N"="N") -> (w64:T20)
                n28 = call "MFLI controller -- via frontend -- V2.vi"("MFLI controller action"=MFLI_controller_action."Scan frequency", "sweep parameters"=w64, "delay (msec)"=w54) -> ("Freq out (Hz)"=w70:dbl[], "sweep time"=→"sweep time (sec)":dbl, "Voltage out (V)"=w69:cdb[])  [unwired: 10 in]
                n29 = flat-sequence {
                  tunnel: w70 -> [w78]
                  tunnel: [w78] -> w60
                  tunnel: w74 -> [w76]
                  tunnel: w69 -> [w75]
                  tunnel: [w75] -> w55
                  frame #0 {
                    n30 = Generate User Event(user event=w76, event data cluster="New sweep data arrives" ("event data")) -> ()  [unwired: 2 in, 2 out]
                  }
                }
                n31 = Delete From Array(array=w60, length=1, index=0) -> (array with subset deleted=→"Freq out":dbl[])  [unwired: 1 out]
                n32 = Delete From Array(array=w55, length=1, index=0) -> (array with subset deleted=→"Voltage out":cdb[])  [unwired: 1 out]
              }
            }
          }
          frame "read from disk" {
            n33 = case shown="True" "read from disk" {
              selector: "read from disk" -> [_ w91]
              tunnel: w82 -> [_ w92]
              tunnel: w81 -> [_ _]
              tunnel: "read file" -> [_ w88]
              frame False {
              }
              frame True {
                n34 = Not(x=w91) -> (.not. x?=w90:bool)
                n35 = local write "read from disk"(w90) -> ()
                n36 = call "file - read-write - list of lines.vi"("read/write control"=file_--_read-write_control."read", "file path"=w88) -> ("list of lines OUT"=w87:string[])  [unwired: 8 in, 1 out]
                n37 = for {
                  tunnel: w87 -> [w99] mode=indexing
                  tunnel: [w97] -> w86 mode=indexing
                  tunnel: [w94] -> w83 mode=indexing
                  w93 = 0.0
                  n38 = Scan From String(format string="%f%f%f", input string=w99, default 1=w93, default 2=w93, default 3=w93) -> (output 1=w97:dbl, output 2=w96:dbl, output 3=w95:dbl)  [unwired: 2 in, 3 out]